vi "Controle_Manip_Main_GUI_Backup2.vi"() -> ()   [LabVIEW 2019] (continued)
          w103 = ""
          # "reset log file and \ncomment to empty"
          # "Build references arrays for real-time update of experiments' indicators"
          n40 = control-ref of="MasterPause"() -> (w60:refnum<vi>)
          n41 = control-ref of="MasterStop"() -> (w57:refnum<vi>)
          n42 = control-ref of="MasterPause"() -> (w58:refnum<vi>)
          n43 = control-ref of="MasterStop"() -> (w59:refnum<vi>)
          n44 = control-ref of="PausePolar"() -> ()  [unwired: 1 out]
          n45 = control-ref of="StopPolar"() -> ()  [unwired: 1 out]
          n46 = control-ref of="XY Intensity Map"() -> (w78:refnum<vi>)
          n47 = control-ref of="CCD 2D Image XY Map"() -> (w79:refnum<vi>)
          n48 = control-ref of="Expected (s)"() -> (w80:refnum<vi>)
          n49 = control-ref of="Elapsed (s)"() -> (w81:refnum<vi>)
          n50 = control-ref of="Scan X Readout (V)"() -> (w75:refnum<vi>)
          n51 = control-ref of="CCD 1D Spectrum XY Map"() -> (w77:refnum<vi>)
          n52 = control-ref of="Stop XY Map"() -> ()  [unwired: 1 out]
          n53 = control-ref of="Scan Y Readout (V)"() -> (w76:refnum<vi>)
          n54 = control-ref of="Scan Main Progess Bar"() -> (w72:refnum<vi>)
          n55 = control-ref of="Save XY Map"() -> (w74:refnum<vi>)
          n56 = control-ref of="Acquire XY Map"() -> (w73:refnum<vi>)
          n57 = control-ref of="KCube Shutter Device Reference"() -> (w90:refnum<vi>)
          n58 = control-ref of="RotStage Exc Angle Readout (°)"() -> (w85:refnum<vi>)
          n59 = control-ref of="RotStage Det Angle Readout (°)"() -> (w86:refnum<vi>)
          n60 = control-ref of="Polarisation 2D Image"() -> (w88:refnum<vi>)
          n61 = control-ref of="Pause XY Map"() -> ()  [unwired: 1 out]
          n62 = control-ref of="Polarisation 1D Spectrum"() -> (w87:refnum<vi>)
          n63 = control-ref of="Acquire Polarisation"() -> (w82:refnum<vi>)
          n64 = control-ref of="Scan Main Progess Bar"() -> (w84:refnum<vi>)
          n65 = control-ref of="Cnts"() -> (w70:refnum<vi>)
          n66 = control-ref of="Shutter Ctrls"() -> (w89:refnum<vi>)
          n67 = control-ref of="Save Polarisation"() -> (w83:refnum<vi>)
          n68 = Bundle("Scan Main Progess Bar"=w72, "Acquire XY Map"=w73, "MasterPause"=w58, "MasterStop"=w57, "Save XY Map"=w74, "Scan X Readout (V)"=w75, "Scan Y Readout (V)"=w76, "CCD 1D Spectrum XY Map"=w77, "XY Intensity Map"=w78, "CCD 2D Image XY Map"=w79, "Expected (s)"=w80, "Elapsed (s)"=w81, "Cnts"=w70) -> (→"Scan XY Map References":T31)  [unwired: 1 in]
          n69 = Bundle("Acquire Polarisation"=w82, "Save Polarisation"=w83, "MasterPause"=w60, "MasterStop"=w59, "Scan Main Progess Bar"=w84, "RotStage Exc Angle Readout (°)"=w85, "RotStage Det Angle Readout (°)"=w86, "Polarisation 1D Spectrum"=w87, "Polarisation 2D Image"=w88, "Shutter Ctrls"=w89, "KCube Shutter Device Reference"=w90) -> (→"Scan Polarisation References":T32)  [unwired: 1 in]
          n70 = control-ref of="Contrast Oscillations"() -> (w97:refnum<vi>)
          n71 = control-ref of="Acquire Contrast"() -> (w96:refnum<vi>)
          n72 = control-ref of="Contrast 1D Spectrum"() -> (w98:refnum<vi>)
          n73 = control-ref of="Save Contrast"() -> (w95:refnum<vi>)
          n74 = control-ref of="Att Pos X"() -> (w63:refnum<vi>)
          n75 = control-ref of="Att Pos Y"() -> (w62:refnum<vi>)
          n76 = control-ref of="Att Pos Z"() -> (w64:refnum<vi>)
          n77 = control-ref of="KCube Shutter Device Reference"() -> (w102:refnum<vi>)
          n78 = control-ref of="PZC Position Readout (usteps)"() -> (w101:refnum<vi>)
          n79 = control-ref of="Stop Contrast"() -> (w99:refnum<vi>)
          n80 = control-ref of="Scan Main Progess Bar"() -> (w94:refnum<vi>)
          n81 = control-ref of="Scan Y Readout (V)"() -> (w68:refnum<vi>)
          n82 = control-ref of="Scan X Readout (V)"() -> (w67:refnum<vi>)
          n83 = local write "NewVal"(FALSE ("NewVal")) -> ()
          n84 = control-ref of="Map Marker X Pos"() -> (w66:refnum<vi>)
          n85 = control-ref of="Map Marker Y Pos"() -> (w65:refnum<vi>)
          n86 = control-ref of="Pause Contrast"() -> (w100:refnum<vi>)
          n87 = control-ref of="Shutter Ctrls"() -> (w92:refnum<vi>)
          n88 = Bundle("Shutter Ctrls"=w92, "KCube Shutter Device Reference"=w102, "Scan Main Progess Bar"=w94, "PZC Position Readout (usteps)"=w101, "Pause Contrast"=w100, "Stop Contrast"=w99, "Contrast 1D Spectrum"=w98, "Contrast Oscillations"=w97, "Acquire Contrast"=w96, "Save Contrast"=w95) -> (→"Contrast References":T14)  [unwired: 1 in]
          n89 = Bundle("Scan Y Readout (V)"=w68, "Scan X Readout (V)"=w67, "Map Marker X Pos"=w66, "Map Marker Y Pos"=w65, "Att Pos Z"=w64, "Att Pos X"=w63, "Att Pos Y"=w62) -> (→"Location Parameters":T6)  [unwired: 1 in]
          n90 = local write "Log file"(w103) -> ()
          n91 = local write "Comment"(w103) -> ()
        }
        frame #3 {
          # "Get Experiment Graph Control numbers"
          n92 = control-ref of="Experiment Graph Controls"() -> (w107:refnum<vi>)
          n93 = property class="TabCtl (strict)"(reference=w107) -> ("Pages"=w105:refnum<vi>[])  [unwired: 1 in, 2 out]
          n94 = call "TabVisibility.vi"("Page Visible"=TRUE, "array"=w105, "MyfinalExpGraphCont"=T29."Absorption" ("Experiment Graph Controls")) -> ()  [unwired: 1 in]
        }
      }
    }
    frame #1 {
      # "Initialisation of all the devices?"
      # "Initialisation of devices connections"
      n95 = call "Initialisation prompt"() -> ("Yes please!"=w108:bool)  [unwired: 18 in, 1 out]
      "Initialise all devices?" <- w108
      n96 = case shown="True" w108 {
        frame False {
          # "Do not activate devices"
          n97 = control-ref of="Tab Objective Sample"() -> (w115:refnum<vi>)
          n98 = property on="Experimental parameters tab" class="TabCtl (strict)" props=["Pages", "Value"]() -> ("Pages"=w117:refnum<vi>[])  [unwired: 2 in, 3 out]
          n99 = property class="TabCtl (strict)"(reference=w115) -> ("Pages"=w113:refnum<vi>[])  [unwired: 1 in, 2 out]
          n100 = property on="Experiment Graph Controls" class="TabCtl (strict)" props=["Value", "Pages"]() -> ("Pages"=w119:refnum<vi>[])  [unwired: 2 in, 3 out]
          n101 = Array Size(array=w113) -> (size(s)=w114:i32)
          n102 = Array Size(array=w117) -> (size(s)=w116:i32)
          n103 = for {
            N: w116 -> [_]
            tunnel: w117 -> [w126]
            i -> [w124]
            n104 = Index Array(array=w126, index=w124) -> (element=w127:refnum<vi>)
            n105 = property class="Page"(reference=w127, "PageVis"=TRUE ("Page Visible")) -> ()  [unwired: 1 in, 2 out]
          }
          n106 = for {
            N: w114 -> [_]
            tunnel: w113 -> [w123]
            i -> [w122]
            n107 = Index Array(array=w123, index=w122) -> (element=w121:refnum<vi>)
            n108 = property class="Page"(reference=w121, "PageVis"=TRUE ("Page Visible")) -> ()  [unwired: 1 in, 2 out]
          }
          n109 = Array Size(array=w119) -> (size(s)=w118:i32)
          n110 = for {
            N: w118 -> [_]
            tunnel: w119 -> [w130]
            i -> [w128]
            n111 = Index Array(array=w130, index=w128) -> (element=w131:refnum<vi>)
            n112 = property class="Page"(reference=w131, "PageVis"=TRUE ("Page Visible")) -> ()  [unwired: 1 in, 2 out]
          }
          n113 = local read "Log file"() -> (w111:string)
          n114 = call "Write2LogFile.vi"("Add to log file"="Initialisation ...\nNo instruments activated.", "Log file before"=w111, "Checkbox"=FALSE) -> ("Log file after"=w112:string)
          n115 = local write "Log file"(w112) -> ()
        }
        frame True {
          # "Activate all the devices selected in the Settings tab"
          n116 = stacked-sequence {
            frame #0 {
              n117 = local read "ESP 301 On?"() -> (w140:bool)
              n118 = local read "ESP 300 On?"() -> (w141:bool)
              n119 = local read "PZC200 On?"() -> (w134:bool)
              n120 = local write "Scan Main Progess Bar"(u8 0 ("Scan Main Progess Bar")) -> ()
              n121 = local read "KCube Shutter On?"() -> (w138:bool)
              n122 = local read "KCubes Piezo On?"() -> (w137:bool)
              n123 = local read "Laser Comm On?"() -> (w132:bool)
              n124 = local read "Cryostation On?"() -> (w142:bool)
              n125 = local read "Attocubes On?"() -> (w143:bool)
              n126 = local read "PM16-120 On?"() -> (w135:bool)
              n127 = local read "LightField On?"() -> (w136:bool)
              n128 = local read "PicoHarp On?"() -> (w133:bool)
              n129 = local read "FSM 300 On?"() -> (w139:bool)
              n130 = global write "InstrumentsOn.vi" "ESP 301 On?"(w140) -> ()
              n131 = global write "InstrumentsOn.vi" "ESP 300 On?"(w141) -> ()
              n132 = global write "InstrumentsOn.vi" "PZC200 On?"(w134) -> ()
              n133 = global write "InstrumentsOn.vi" "Attocubes On?"(w143) -> ()
              n134 = global write "InstrumentsOn.vi" "Cryostation On?"(w142) -> ()
              n135 = global write "InstrumentsOn.vi" "PM16-120 On?"(w135) -> ()
              n136 = global write "InstrumentsOn.vi" "LightField On?"(w136) -> ()
              n137 = global write "InstrumentsOn.vi" "Laser Comm On?"(w132) -> ()
              n138 = global write "InstrumentsOn.vi" "KCubes Piezo On?"(w137) -> ()
              n139 = global write "InstrumentsOn.vi" "KCube Shutter On?"(w138) -> ()
              n140 = global write "InstrumentsOn.vi" "FSM 300 On?"(w139) -> ()
              n141 = global write "InstrumentsOn.vi" "PicoHarp On?"(w133) -> ()
            }
            frame #1 {
              # "LLTF"
              n142 = case shown="True" "LLTF On?" {
                frame False {
                }
                frame True {
                  n143 = Automation Open(Automation Refnum="xphyspecLib.IXPhySpec") -> (Automation Refnum=w163:refnum<k7>, error out=w162:errorcluster)  [unwired: 3 in]
                  n144 = local read "Excitation Wavelength (nm)"() -> (w153:dbl)
                  n145 = call "newinit.vi"("error in"=w162, "Automation Refnum"=w163) -> ("error out"=w159:errorcluster, "Detected?"=→"LLTF Detected?":bool, "xphyspecLib.IXPhySpec out"=w160:refnum<k7>)  [unwired: 7 in]
                  n146 = call "listandgetdeviceinterface.vi"("error in (no error)"=w159, "reference"=w160) -> ("LLTF error out"=→"LLTFDevice error out":errorcluster, "LLTFDevice Interface"=w155:refnum<k7>, "error out to close"=→"LLTF Error":errorcluster, "reference out to lose"=→"LLTF Reference":refnum<k7>)  [unwired: 6 in]
                  n147 = call "testmove.vi"("p_TargetWavelength"=w153, "reference"=w155) -> ("CurrentWavelength"=→"CurrentWL":dbl, "CurrentAngle"=→"CurrentAngle":dbl, "Device reference out"=→"LLTFDevice Interface":refnum<k7>, "Device moved"=→"Device moved":bool)  [unwired: 4 in, 2 out]
                  n148 = local read "Log file"() -> (w149:string)
                  n149 = call "Write2LogFile.vi"("Add to log file"="Initialise communication with PhotonEtc LLTF", "Log file before"=w149, "Checkbox"=FALSE) -> ("Log file after"=w148:string)
                  n150 = local write "Log file"(w148) -> ()
                }
              }
            }
            frame #2 {
              # "ESP 300: 1 Jobin Yvon 320 Monochromator"
              n151 = control-ref of="CCD 1D Spectrum Main  Cursor2WL 1 Mono 2"() -> (w167:refnum<vi>)
              n152 = control-ref of="CCD 1D Spectrum Main  Cursor2WL 2 Mono 2"() -> (w166:refnum<vi>)
              n153 = local read "ESP300 COM Port"() -> (w165:refnum<visa-resource-name>)
              n154 = case shown="True" "ESP 300 On?" {
                tunnel: [enum16{"Enabled", "Disabled", "Disabled&Grayed"}."Disabled&Grayed" ("Enum") enum16{"Enabled", "Disabled", "Disabled&Grayed"}."Enabled" ("Enum")] -> w169
                tunnel: w165 -> [w174 w177]
                frame False {
                  n155 = global write "InstrumentReferences.vi" "ESP300 COM Port"(w174) -> ()
                }
                frame True {
                  n156 = global write "InstrumentReferences.vi" "ESP300 COM Port"(w177) -> ()
                  n157 = control-ref of="Mono2 Velocity"() -> (w181:refnum<vi>)
                  n158 = control-ref of="Mono2 Motor Pos"() -> (w180:refnum<vi>)
                  n159 = call "subVI_Init&GetParams.vi"("Mono2 Pos"=w180, "Mono2 Velocity"=w181) -> ("Mono2 On"=w182:bool)  [unwired: 1 in]
                  n160 = local read "Log file"() -> (w186:string)
                  n161 = local write "Mono2 On"(w182) -> ()
                  n162 = call "Write2LogFile.vi"("Add to log file"="Initialise communication with ESP 300", "Log file before"=w186, "Checkbox"=FALSE) -> ("Log file after"=w185:string)
                  n163 = local write "Log file"(w185) -> ()
                  n164 = control-ref of="Mono2 Wavelength (nm)"() -> (w179:refnum<vi>)
                  n165 = property class="DigNum (strict)"(reference=w179, "DisabledEnum"=T28."Disabled and Grayed Out" ("Disabled")) -> ()  [unwired: 1 in, 2 out]
                }
              }
              n166 = control-ref of="Mono2 On"() -> (w170:refnum<vi>)
              n167 = control-ref of="Mono2 Wavelength (nm)"() -> (w171:refnum<vi>)
              n168 = control-ref of="Mono2 Motor Pos"() -> (w168:refnum<vi>)
              n169 = Build Array(w170, w171, w168, w167, w166) -> (w172:refnum<vi>[])
              n170 = call "Enable&Disable_Controls.vi"("Enum"=w169, "References"=w172) -> ()  [unwired: 1 in]
            }
            frame #3 {
              # "ESP 301: 2 rotation stages + 1 linear translation stage"
              n171 = case shown="True" "ESP 301 On?" {
                frame False {
                  n172 = control-ref of="Experiment Graph Controls"() -> (w190:refnum<vi>)
                  n173 = local read "Scan Polar AllParams"() -> (w202:refnum<vi>[])
                  n174 = property class="TabCtl (strict)"(reference=w190) -> ("Pages"=w194:refnum<vi>[])  [unwired: 1 in, 2 out]
                  n175 = property class="TabCtl (strict)"(reference=w190) -> ("Pages"=w191:refnum<vi>[])  [unwired: 1 in, 2 out]
                  n176 = call "Enable&Disable_Controls.vi"("Enum"=enum16{"Enabled", "Disabled", "Disabled&Grayed"}."Disabled&Grayed", "References"=w202) -> ()  [unwired: 1 in]
                  n177 = property on="Experimental parameters tab" class="TabCtl (strict)"() -> ("Pages"=w197:refnum<vi>[])  [unwired: 2 in, 2 out]
                  n178 = call "TabVisibility.vi"("Page Visible"=FALSE, "array"=w194, "MyfinalExpGraphCont"=T29."Polarisation Acquisition") -> ()  [unwired: 1 in]
                  n179 = call "TabVisibility.vi"("Page Visible"=FALSE, "array"=w191, "MyfinalExpGraphCont"=T29."Contrast Acquisition") -> ()  [unwired: 1 in]
                  n180 = local read "Scan Translation Coarse Ctrls"() -> (w196:refnum<vi>[])
                  n181 = Index Array(array=w197, index=2) -> (element=w204:refnum<vi>)
                  n182 = Index Array(array=w197, index=3) -> (element=w198:refnum<vi>)
                  n183 = property class="Page"(reference=w198, "PageVis"=FALSE ("Page Visible")) -> ()  [unwired: 1 in, 2 out]
                  n184 = property class="Page"(reference=w204, "PageVis"=FALSE ("Page Visible")) -> ()  [unwired: 1 in, 2 out]
                  n185 = call "Enable&Disable_Controls.vi"("Enum"=enum16{"Enabled", "Disabled", "Disabled&Grayed"}."Disabled&Grayed", "References"=w196) -> ()  [unwired: 1 in]
                }
                frame True {
                  n186 = stacked-sequence {
                    frame #0 {
                      n187 = local read "Log file"() -> (w209:string)
                      n188 = call "Write2LogFile.vi"("Add to log file"="Initialise communication with ESP 301", "Log file before"=w209, "Checkbox"=FALSE) -> ("Log file after"=w207:string)
                      n189 = local write "Log file"(w207) -> ()
                    }
                    frame #1 {
                      n190 = control-ref of="Experiment Graph Controls"() -> (w216:refnum<vi>)
                      n191 = property class="TabCtl (strict)"(reference=w216) -> ("Pages"=w217:refnum<vi>[])  [unwired: 1 in, 2 out]
                      n192 = property on="Experimental parameters tab" class="TabCtl (strict)"("Value"=T19."Polarisation" ("Experimental parameters tab")) -> ("Pages"=w222:refnum<vi>[])  [unwired: 2 in, 2 out]
                      n193 = property on="Experimental parameters tab" class="TabCtl (strict)"() -> ("Pages"=w229:refnum<vi>[])  [unwired: 2 in, 2 out]
                      n194 = property class="TabCtl (strict)"(reference=w216) -> ("Pages"=w220:refnum<vi>[])  [unwired: 1 in, 2 out]
                      n195 = call "TabVisibility.vi"("Page Visible"=TRUE, "array"=w217, "MyfinalExpGraphCont"=T29."Contrast Acquisition") -> ()  [unwired: 1 in]
                      n196 = Index Array(array=w222, index=3) -> (element=w225:refnum<vi>)
                      n197 = Index Array(array=w229, index=2) -> (element=w226:refnum<vi>)
                      n198 = call "TabVisibility.vi"("Page Visible"=TRUE, "array"=w220, "MyfinalExpGraphCont"=T29."Polarisation Acquisition") -> ()  [unwired: 1 in]
                      n199 = property class="Page"(reference=w226, "PageVis"=TRUE ("Page Visible")) -> ()  [unwired: 1 in, 2 out]
                      n200 = property class="Page"(reference=w225, "PageVis"=TRUE ("Page Visible")) -> ()  [unwired: 1 in, 2 out]
                      n201 = local read "Scan Translation Coarse Ctrls"() -> (w215:refnum<vi>[])
                      n202 = local read "Scan Polar AllParams"() -> (w213:refnum<vi>[])
                      n203 = call "Enable&Disable_Controls.vi"("Enum"=enum16{"Enabled", "Disabled", "Disabled&Grayed"}."Enabled", "References"=w215) -> ()  [unwired: 1 in]
                      n204 = call "Enable&Disable_Controls.vi"("Enum"=enum16{"Enabled", "Disabled", "Disabled&Grayed"}."Enabled", "References"=w213) -> ()  [unwired: 1 in]
                    }
                    frame #2 {
                      n205 = flat-sequence {
                        tunnel: [w236] -> w230
                        frame #0 {
                          w236 = refnum<visa-resource-name> "COM8" ("ESP 301 COM Port")
                          n206 = call "Close.vi"("VISA resource name"=w236) -> ()  [unwired: 10 in, 1 out]
                        }
                        frame #1 {
                          n207 = call "_Create Instrument Channel_libESP301.vi"("COM Port (1)"=u16 8) -> ()  [unwired: 8 in, 3 out]
                        }
                      }
                      n208 = call "Initialize.vi"("VISA resource name"=w230, "ID Query (True)"=TRUE, "Reset (False)"=FALSE ("ID Query (True)"), "Serial Link (RS232)"=enum16{"RS232", "USB"}."USB") -> ("VISA resource name out"=w231:refnum<visa-resource-name>, "error out"=w235:errorcluster)  [unwired: 5 in]
                      n209 = case shown="Default" w235 {
                        tunnel: w231 -> [_ _]
                        frame No Error {
                        }
                        frame Default {
                          w243 = FALSE ("ID Query (True)")
                          n210 = call "Connect Newport Instruments_libESP301.vi"() -> ("error (duplicate)"=w241:errorcluster, "VISA resource name (duplicate)"=w238:refnum<visa-resource-name>)  [unwired: 7 in, 3 out]
                          n211 = call "_Close Communications_libESP301.vi"("Instrument Channel"=w238, "error in (no error)"=w241) -> ("error out"=w240:errorcluster)  [unwired: 13 in]
                          n212 = call "Initialize.vi"("VISA resource name"=w238, "ID Query (True)"=w243, "Reset (False)"=w243, "error in (no error)"=w240, "Serial Link (RS232)"=enum16{"RS232", "USB"}."USB") -> ("VISA resource name out"=w239:refnum<visa-resource-name>)  [unwired: 4 in, 1 out]
                          n213 = local write "ESP 301 COM Port"(w239) -> ()
                        }
                      }
                      n214 = local write "ESP 301 COM Port"(w231) -> ()
                    }
                    frame #3 {
                      # "Initialise ESP301 communication\nand motor parameters & limits"
                      n215 = local read "ESP 301 COM Port"() -> (w244:refnum<visa-resource-name>)
                      n216 = for {
                        N: 3 -> [_]
                        tunnel: w244 -> [w257]
                        tunnel: [w256] -> _
                        i -> [w247]
                        n217 = Increment(x=w247) -> (x+1=w246:i32)
                        n218 = call "Get Left Travel Limit.vi"("Axis (1)"=w246, "VISA resource name"=w257) -> ("Left Travel Limit (units)"=w253:dbl, "VISA resource name out"=w260:refnum<visa-resource-name>)  [unwired: 3 in, 1 out]
                        n219 = call "Get Right Travel Limit.vi"("Axis (1)"=w246, "VISA resource name"=w260) -> ("Right Travel Limit (units)"=w252:dbl, "VISA resource name out"=w259:refnum<visa-resource-name>)  [unwired: 3 in, 1 out]
                        n220 = call "Get Velocity.vi"("Axis (1)"=w246, "VISA resource name"=w259) -> ("Velocity (units/s)"=w251:dbl, "VISA resource name out"=w258:refnum<visa-resource-name>)  [unwired: 3 in, 1 out]
                        n221 = call "Read Actual Position.vi"("Axis (1)"=w246, "VISA resource name"=w258) -> ("Position (units)"=w248:dbl, "VISA resource name out"=w255:refnum<visa-resource-name>)  [unwired: 3 in, 1 out]
                        n222 = call "Get Maximum Velocity.vi"("Axis (1)"=w246, "VISA resource name"=w255) -> ("Maximum Velocity (units/s)"=w250:dbl, "VISA resource name out"=w254:refnum<visa-resource-name>)  [unwired: 3 in, 1 out]
                        n223 = call "Get Motor Power Status.vi"("Axis (1)"=w246, "VISA resource name"=w254) -> ("Power Status"=w249:bool, "VISA resource name out"=w256:refnum<visa-resource-name>)  [unwired: 3 in, 1 out]
                        n224 = case shown="1" w246 {
                          tunnel: w253 -> [_ w266 w272 w278]
                          tunnel: w252 -> [_ w265 w271 w277]
                          tunnel: w251 -> [_ w264 w270 w275]
                          tunnel: w250 -> [_ w263 w268 w276]
                          tunnel: w249 -> [_ w262 w267 w273]
                          tunnel: w248 -> [_ w261 w269 w274]
                          frame 0, Default {
                          }
                          frame 1 {
                            # "Translation stage"
                            n225 = property on="Newport Linear Translation Stage Position (mm)" class="DigNum (strict)"("Minimum"=w266, "Maximum"=w265) -> ()  [unwired: 2 in, 2 out]
                            n226 = local write "Newport Linear Translation Stage Velocity (mm/s)"(w264) -> ()
                            n227 = local write "Newport Linear Translation Stage Position Readout (mm)"(w261) -> ()
                            n228 = property on="Newport Linear Translation Stage Velocity (mm/s)" class="DigNum (strict)"("Maximum"=w263) -> ()  [unwired: 2 in, 2 out]
                            n229 = local write "Motor LinT On?"(w262) -> ()
                          }
                          frame 2 {
                            # "RotStage Det"
                            n230 = property on="RotStage Det Angle (°)" class="DigNum (strict)"("Maximum"=w272, "Minimum"=w271) -> ()  [unwired: 2 in, 2 out]
                            n231 = local write "RotStage Det Velocity (°/s)"(w270) -> ()
                            n232 = property on="RotStage Det Velocity (°/s)" class="DigNum (strict)"("Maximum"=w268) -> ()  [unwired: 2 in, 2 out]
                            n233 = local write "RotStage Det Angle Readout (°)"(w269) -> ()
                            n234 = local write "Motor RotStage Det On?"(w267) -> ()
                          }
                          frame 3 {
                            # "RotStage Exc"
                            n235 = property on="RotStage Exc Angle (°)" class="DigNum (strict)"("Maximum"=w278, "Minimum"=w277) -> ()  [unwired: 2 in, 2 out]
                            n236 = local write "RotStage Exc Velocity (°/s)"(w275) -> ()
                            n237 = property on="RotStage Exc Velocity (°/s)" class="DigNum (strict)"("Maximum"=w276) -> ()  [unwired: 2 in, 2 out]
                            n238 = local write "RotStage Exc Angle Readout (°)"(w274) -> ()
                            n239 = local write "Motor RotStage Exc On?"(w273) -> ()
                          }
                        }
                      }
                    }
                    frame #4 {
                      n240 = local read "ESP 301 COM Port"() -> (w279:refnum<visa-resource-name>)
                      n241 = call "Get Motor Power Status.vi"("Axis (1)"=1, "VISA resource name"=w279) -> ("error out"=w286:errorcluster, "Power Status"=w282:bool, "VISA resource name out"=w287:refnum<visa-resource-name>)  [unwired: 3 in]
                      n242 = local write "Motor LinT On?"(w282) -> ()
                      n243 = call "Get Motor Power Status.vi"("error in (no error)"=w286, "Axis (1)"=2, "VISA resource name"=w287) -> ("error out"=w289:errorcluster, "Power Status"=w280:bool, "VISA resource name out"=w288:refnum<visa-resource-name>)  [unwired: 2 in]
                      n244 = local write "Motor RotStage Exc On?"(w280) -> ()
                      n245 = call "Get Motor Power Status.vi"("error in (no error)"=w289, "Axis (1)"=3, "VISA resource name"=w288) -> ("error out"=w290:errorcluster, "Power Status"=w281:bool)  [unwired: 2 in, 1 out]
                      n246 = local write "Motor RotStage Det On?"(w281) -> ()
                      n247 = local write "ESP 301 Error"(w290) -> ()
                    }
                  }
                }
              }
            }
            frame #4 {
              # "Advance progress bar"
              n248 = local write "Scan Main Progess Bar"(u8 5 ("Scan Main Progess Bar")) -> ()
            }
            frame #5 {
              # "LightField: Monochromator SpectraPro HRS-500 + CCD Pixis"
              n249 = case shown="True" "LightField On?" {
                frame False {
                  n250 = control-ref of="Grating"() -> (w306:refnum<vi>)
                  n251 = control-ref of="Center Wavelength (nm)"() -> (w308:refnum<vi>)
                  n252 = local read "PicoHarp On?"() -> (w314:bool)
                  n253 = local read "ESP 300 On?"() -> (w315:bool)
                  n254 = control-ref of="Accumulations"() -> (w311:refnum<vi>)
                  n255 = control-ref of="CCD ROI"() -> (w310:refnum<vi>)
                  n256 = control-ref of="Exposure Time (ms)"() -> (w309:refnum<vi>)
                  n257 = control-ref of="Exit mirror"() -> (w307:refnum<vi>)
                  n258 = And(x=w315, y=w314) -> (x .and. y?=w313:bool)
                  n259 = case shown="False" w313 {
                    frame False {
                      n260 = control-ref of="Experiment Graph Controls"() -> (w317:refnum<vi>)
                      n261 = property class="TabCtl (strict)"(reference=w317) -> ("Pages"=w319:refnum<vi>[])  [unwired: 1 in, 2 out]
                      n262 = call "TabVisibility.vi"("Page Visible"=FALSE, "array"=w319, "MyfinalExpGraphCont"=T29."Spectrum Acquisition") -> ()  [unwired: 1 in]
                    }
                    frame True {
                      n263 = control-ref of="Experiment Graph Controls"() -> (w321:refnum<vi>)
                      n264 = property class="TabCtl (strict)"(reference=w321) -> ("Pages"=w323:refnum<vi>[])  [unwired: 1 in, 2 out]
                      n265 = call "TabVisibility.vi"("Page Visible"=TRUE, "array"=w323, "MyfinalExpGraphCont"=T29."Spectrum Acquisition") -> ()  [unwired: 1 in]
                    }
                  }
                  n266 = Build Array(w308, w307, w306, w311, w310, w309) -> (w312:refnum<vi>[])
                  n267 = call "Enable&Disable_Controls.vi"("Enum"=enum16{"Enabled", "Disabled", "Disabled&Grayed"}."Disabled&Grayed", "References"=w312) -> ()  [unwired: 1 in]
                  n268 = control-ref of="Experiment Graph Controls"() -> (w304:refnum<vi>)
                  n269 = control-ref of="Experiment Graph Controls"() -> (w299:refnum<vi>)
                  n270 = control-ref of="Experiment Graph Controls"() -> (w298:refnum<vi>)
                  n271 = property class="TabCtl (strict)"(reference=w304) -> ("Pages"=w302:refnum<vi>[])  [unwired: 1 in, 2 out]
                  n272 = property class="TabCtl (strict)"(reference=w299) -> ("Pages"=w301:refnum<vi>[])  [unwired: 1 in, 2 out]
                  n273 = property class="TabCtl (strict)"(reference=w298) -> ("Pages"=w296:refnum<vi>[])  [unwired: 1 in, 2 out]
                  n274 = call "TabVisibility.vi"("Page Visible"=FALSE, "array"=w302, "MyfinalExpGraphCont"=T29."Intensity Map Acquisition") -> ()  [unwired: 1 in]
                  n275 = call "TabVisibility.vi"("Page Visible"=FALSE, "array"=w301, "MyfinalExpGraphCont"=T29."Polarisation Acquisition") -> ()  [unwired: 1 in]
                  n276 = call "TabVisibility.vi"("Page Visible"=FALSE, "array"=w296, "MyfinalExpGraphCont"=T29."Contrast Acquisition") -> ()  [unwired: 1 in]
                }
                frame True {
                  n277 = stacked-sequence {
                    seq-local: [_ _ "uPL" ("ExperimentName") _ _ _ _] -> [_ _ _ w354 _ _ _]
                    seq-local: [_ _ w348 _ _ _ _] -> [_ _ _ w355 _ _ _]
                    seq-local: [_ _ w347 _ _ _ _] -> [_ _ _ w353 _ _ _]
                    seq-local: [_ _ _ w352 _ _ _] -> [_ _ _ _ w364 _ _]
                    seq-local: [_ _ _ w351 _ _ _] -> [_ _ _ _ w363 _ _]
                    seq-local: [_ _ _ _ w358 _ _] -> [_ _ _ _ _ w371 _]
                    seq-local: [_ _ _ _ w359 _ _] -> [_ _ _ _ _ w372 _]
                    seq-local: [_ _ _ _ w357 _ _] -> [_ _ _ _ _ w370 _]
                    frame #0 {
                      n278 = control-ref of="Grating"() -> (w326:refnum<vi>)
                      n279 = control-ref of="Center Wavelength (nm)"() -> (w328:refnum<vi>)
                      n280 = control-ref of="Accumulations"() -> (w331:refnum<vi>)
                      n281 = control-ref of="CCD ROI"() -> (w330:refnum<vi>)
                      n282 = control-ref of="Exposure Time (ms)"() -> (w329:refnum<vi>)
                      n283 = control-ref of="Exit mirror"() -> (w327:refnum<vi>)
                      n284 = local read "Log file"() -> (w334:string)
                      n285 = Build Array(w328, w327, w326, w331, w330, w329) -> (w332:refnum<vi>[])
                      n286 = call "Write2LogFile.vi"("Add to log file"="Launching LightField (~ 20 s)", "Log file before"=w334, "Checkbox"=FALSE) -> ("Log file after"=w335:string)
                      n287 = call "Enable&Disable_Controls.vi"("Enum"=enum16{"Enabled", "Disabled", "Disabled&Grayed"}."Enabled", "References"=w332) -> ()  [unwired: 1 in]
                      n288 = local write "Log file"(w335) -> ()
                    }
                    frame #1 {
                      n289 = control-ref of="Experiment Graph Controls"() -> (w337:refnum<vi>)
                      n290 = control-ref of="Experimental parameters tab"() -> (w341:refnum<vi>)
                      n291 = property class="TabCtl (strict)"(reference=w337) -> ("Pages"=w339:refnum<vi>[])  [unwired: 1 in, 2 out]
                      n292 = property class="TabCtl (strict)"(reference=w341, "Value"=T19."Monochromators & CCD") -> ("Pages"=w344:refnum<vi>[])  [unwired: 1 in, 2 out]
                      n293 = call "TabVisibility.vi"("Page Visible"=TRUE, "array"=w339, "MyfinalExpGraphCont"=T29."Spectrum Acquisition") -> ()  [unwired: 1 in]
                      n294 = Index Array(array=w344, index=0) -> (element=w345:refnum<vi>)
                      n295 = property class="Page"(reference=w345, "PageVis"=TRUE ("Page Visible")) -> ()  [unwired: 1 in, 2 out]
                    }
                    frame #2 {
                      n296 = call "LFA_Initialize.vi"("Is Visible?"="LF Visible") -> ("error out"=w348:errorcluster, "LightField Automation out"=w347:refnum<class "LightField Automation.lvclass">)  [unwired: 9 in]
                    }
                    frame #3 {
                      n297 = local write "Scan Main Progess Bar"(u8 15 ("Scan Main Progess Bar")) -> ()
                      n298 = call "Exp_SetExperiment.vi"("error in (no error)"=w355, "ExperimentName"=w354, "LightField Automation in"=w353) -> ("error out"=w352:errorcluster, "LightField Automation out"=w351:refnum<class "LightField Automation.lvclass">)  [unwired: 7 in]
                    }
                    frame #4 {
                      n299 = local read "Log file"() -> (w362:string)
                      n300 = call "Write2LogFile.vi"("Add to log file"="Getting parameters", "Log file before"=w362, "Checkbox"=FALSE) -> ("Log file after"=w361:string)
                      n301 = local write "Log file"(w361) -> ()
                      n302 = call "Exp_CCD_GetExposureTime.vi"("error in (no error)"=w364, "LightField Automation in"=w363) -> ("error out"=w358:errorcluster, "Exposure Time (s)"=w357:dbl, "LightField Automation out"=w359:refnum<class "LightField Automation.lvclass">)  [unwired: 7 in]
                    }
                    frame #5 {
                      n303 = call "Exp_CCD_GetTemperature.vi"("error in (no error)"=w371, "LightField Automation in"=w372) -> ("error out"=w375:errorcluster, "Temperature (°C)"=→"CCD T° :":dbl, "LightField Automation out"=w374:refnum<class "LightField Automation.lvclass">)  [unwired: 7 in]
                      n304 = call "spec_GetGratings.vi"("error in (no error)"=w375, "LightField Automation in"=w374) -> ("error out"=w383:errorcluster, "Current Grating"=w377:string, "LightField Automation out"=w384:refnum<class "LightField Automation.lvclass">)  [unwired: 6 in, 1 out]
                      n305 = call "spec_GetCenterWavelength.vi"("error in (no error)"=w383, "LightField Automation in"=w384) -> ("error out"=w381:errorcluster, "Center Wavelength"=w378:dbl, "LightField Automation out"=w380:refnum<class "LightField Automation.lvclass">)  [unwired: 7 in]
                      n306 = local write "Grating"(w377) -> ()
                      n307 = call "spec_getCalibration.vi"("error in (no error)"=w381, "LightField Automation in"=w380) -> ("error out"=w368:errorcluster, "ColumnCalibration"=→"Wavelength calibration":dbl[], "LightField Automation out"=w369:refnum<class "LightField Automation.lvclass">)  [unwired: 7 in]
                      n308 = call "spec_GetOpticalExitPort.vi"("error in (no error)"=w368, "LightField Automation in"=w369) -> ("error out"=w367:errorcluster, "Exit Port Location"=w366:T33, "LightField Automation out"=w365:refnum<class "LightField Automation.lvclass">)  [unwired: 7 in]
                      n309 = local write "Center Wavelength (nm)"(w378) -> ()
                      n310 = global write "InstrumentReferences.vi" "LightField Automation out"(w365) -> ()
                      n311 = local write "LightField Automation out"(w365) -> ()
                      n312 = local write "LightField Automation error out"(w367) -> ()
                      n313 = local write "Exit mirror"(w366) -> ()
                      n314 = Multiply(x=w370, y=1000.0) -> (x*y=w379:dbl)
                      n315 = local write "Exposure Time (ms)"(w379) -> ()
                      n316 = local write "Acq Time (ms)"(w379) -> ()
                    }
                    frame #6 {
                      n317 = local write "Scan Main Progess Bar"(u8 35 ("Scan Main Progess Bar")) -> ()
                    }
                  }
                }
              }
            }
            frame #6 {
              # "Thorlabs USB photodiode"
              n318 = case shown="True" "PM16-120 On?" {
                frame False {
                  n319 = property on="Excitation Power (uW)" class="DigNum (strict)"("Label.BG Color"=u32 16711680 ("Label.Colors:BG Color")) -> ()  [unwired: 2 in, 2 out]
                }
                frame True {
                  w389 = refnum<visa-resource-name> "USB0::0x1313::0x807B::190927109::INSTR" ("instrument handle")
                  # "Initialise powermeter"
                  n320 = call <instrlib>:"TLPM Find Resources.vi"("instrument handle"=w389) -> ("error out"=w394:errorcluster, "Resource Count"=w396:u32)  [unwired: 8 in, 1 out]
                  n321 = property on="Excitation Power (uW)" class="DigNum (strict)"("Blinking"=FALSE) -> ()  [unwired: 2 in, 2 out]
                  n322 = Greater Or Equal?(x=w396, y=1) -> (x >= y?=w395:bool)
                  n323 = case shown="True" w395 {
                    tunnel: w394 -> [_ w409]
                    tunnel: w389 -> [w401 w402]
                    frame False {
                      w400 = FALSE ("ID Query (Do Query)")
                      n324 = call <instrlib>:"TLPM Initialize.vi"("Reset Device (Reset Device)"=w400, "ID Query (Do Query)"=w400, "resource name"=w401) -> ("error out"=w398:errorcluster, "instrument handle out"=w399:refnum<visa-resource-name>)  [unwired: 7 in]
                      n325 = local write "Photodiode handle out"(w399) -> ()
                      n326 = local write "Photodiode error out"(w398) -> ()
                    }
                    frame True {
                      w408 = FALSE ("Reset Device (Reset Device)")
                      # "Select first Device\n(Device Index 0)"
                      n327 = call <instrlib>:"TLPM Get Resource Name.vi"("error in (no error)"=w409, "Index (0)"=u32 0) -> ("error out"=w407:errorcluster)  [unwired: 7 in, 2 out]
                      n328 = local write "Photodiode Status"(TRUE) -> ()
                      n329 = call <instrlib>:"TLPM Initialize.vi"("error in (no error)"=w407, "Reset Device (Reset Device)"=w408, "ID Query (Do Query)"=w408, "resource name"=w402) -> ("error out"=w404:errorcluster, "instrument handle out"=w405:refnum<visa-resource-name>)  [unwired: 6 in]
                      n330 = local write "Photodiode handle out"(w405) -> ()
                      n331 = local write "Photodiode error out"(w404) -> ()
                    }
                  }
                  n332 = local read "Log file"() -> (w393:string)
                  n333 = call "Write2LogFile.vi"("Add to log file"="Initialise communication with Photodiode", "Log file before"=w393, "Checkbox"=FALSE) -> ("Log file after"=w392:string)
                  n334 = local write "Log file"(w392) -> ()
                }
              }
            }
            frame #7 {
              # "448.3nm Laser Diode + Temp Controller & Driver"
              n335 = case shown="True" "Laser Comm On?" {
                frame False {
                  w411 = FALSE ("Visible")
                  n336 = property on="TEC Output" class="Bool (strict)"("Visible"=w411) -> ()  [unwired: 2 in, 2 out]
                  n337 = property on="TEC Temperature" class="DigNum (strict)"("Visible"=w411) -> ()  [unwired: 2 in, 2 out]
                  n338 = property on="Laser Diode Current Set" class="Slide (strict)"("Visible"=w411) -> ()  [unwired: 2 in, 2 out]
                  n339 = property on="Laser on? Control" class="Bool (strict)"("Visible"=w411) -> ()  [unwired: 2 in, 2 out]
                }
                frame True {
                  n340 = local read "Log file"() -> (w415:string)
                  n341 = call "Write2LogFile.vi"("Add to log file"="Initialise communication with Laser Driver", "Log file before"=w415, "Checkbox"=FALSE) -> ("Log file after"=w414:string)
                  n342 = local write "Log file"(w414) -> ()
                  n343 = call "LaserDiodeInit.vi"("resource name"=refnum<visa-resource-name> "USB0::0x1313::0x804F::M00549740::INSTR" ("Diode Driver COM")) -> ("Diode Driver Error"=w420:errorcluster, "Temperature"=w417:dbl, "TEC Output"=w419:bool, "resource out"=→"DDE":refnum<visa-resource-name>, "LD Output"=w418:bool, "Serial Number"=→"Serial Number":string)
                  n344 = local write "Laser on?"(w418) -> ()
                  n345 = local write "Laser on? Control"(w418) -> ()
                  n346 = local write "TEC Output"(w419) -> ()
                  n347 = local write "TEC Temperature"(w417) -> ()
                  n348 = local write "Diode Driver Error"(w420) -> ()
                  n349 = property on="Laser Diode Current Set" class="Slide (strict)"("Visible"=w419) -> ()  [unwired: 2 in, 2 out]
                  n350 = property on="Laser Safety" class="Ring (strict)"("Visible"=w419) -> ()  [unwired: 2 in, 2 out]
                  n351 = property on="Laser on? Control" class="Bool (strict)"("Visible"=w419) -> ()  [unwired: 2 in, 2 out]
                }
              }
            }
            frame #8 {
              # "Excitation wavelength"
              n352 = disable-structure shown="Enabled" {
                disable-tunnel: [w426 458.3] -> w425
                frame Disabled {
                  n353 = call "PromptUserWavelength_DefautValue.vi"() -> ("Wavelength"=w426:dbl)  [unwired: 17 in, 2 out]
                }
                frame Enabled {
                }
              }
              n354 = call "nm2WL.vi"("Wavelength (380 - 780)"=w425) -> ("Color"=w423:u32, "Out Of Range"=w424:bool)
              n355 = case shown="False" w424 {
                tunnel: w423 -> [w431 _]
                frame False {
                  # "set laser color"
                  n356 = Bundle("Color"=w431, "Color"=w431) -> (w430:cluster{"Color":u32, "Color":u32})  [unwired: 1 in]
                  n357 = Bundle(u32 16777216, u32 16777216) -> (w429:cluster{u32, u32})  [unwired: 1 in]
                  n358 = Build Array(w429, w430) -> (w428:cluster{"Color":u32, "Color":u32}[])
                  n359 = property on="Laser on?" class="Bool (strict)"("Colors [4]"=w428) -> ()  [unwired: 2 in, 2 out]
                }
                frame True {
                }
              }
              n360 = local write "Excitation Wavelength (nm)"(w425) -> ()
            }
            frame #9 {
              # "Advancec progress bar"
              n361 = local write "Scan Main Progess Bar"(u8 50 ("Scan Main Progess Bar")) -> ()
            }
            frame #10 {
              # "FSM"
              n362 = local read "FSM 300 On?"() -> (w435:bool)
              n363 = case shown="True" w435 {
                frame True {
                  n364 = stacked-sequence {
                    frame #0 {
                      n365 = local read "Log file"() -> (w439:string)
                      n366 = call "Write2LogFile.vi"("Add to log file"="Initialise communication with FSM", "Log file before"=w439, "Checkbox"=FALSE) -> ("Log file after"=w438:string)
                      n367 = local write "Log file"(w438) -> ()
                    }
                    frame #1 {
                      n368 = control-ref of="Experiment Graph Controls"() -> (w440:refnum<vi>)
                      n369 = property on="Experimental parameters tab" class="TabCtl (strict)"("Value"=T19."Steering mirror" ("Experimental parameters tab")) -> ("Pages"=w448:refnum<vi>[])  [unwired: 2 in, 2 out]
                      n370 = property class="TabCtl (strict)"(reference=w440) -> ("Pages"=w442:refnum<vi>[])  [unwired: 1 in, 2 out]
                      n371 = Index Array(array=w448, index=1) -> (element=w446:refnum<vi>)
                      n372 = property class="Page"(reference=w446, "PageVis"=TRUE ("Page Visible")) -> ()  [unwired: 1 in, 2 out]
                      n373 = call "TabVisibility.vi"("Page Visible"=TRUE, "array"=w442, "MyfinalExpGraphCont"=T29."Intensity Map Acquisition" ("Experiment Graph Controls")) -> ()  [unwired: 1 in]
                    }
                    frame #2 {
                      w453 = 10.0 ("maximum value")
                      w455 = 10.0 ("maximum value")
                      n374 = local read "FSM Y Axis"() -> (w451:tag)
                      n375 = local read "FSM X Axis"() -> (w454:tag)
                      n376 = Negate(x=w455) -> (-x=w456:dbl)
                      n377 = Negate(x=w453) -> (-x=w452:dbl)
                      n378 = call-poly <vilib>:"DAQmx Create Virtual Channel.vi"("maximum value"=w455, "minimum value"=w456, "physical channels"=w454) -> ("task out"=→"FSM X Task":refnum<k21>)  [unwired: 11 in, 1 out]
                      n379 = call-poly <vilib>:"DAQmx Create Virtual Channel.vi"("maximum value"=w453, "minimum value"=w452, "physical channels"=w451) -> ("task out"=→"FSM Y Task":refnum<k21>)  [unwired: 11 in, 1 out]
                    }
                  }
                }
                frame False {
                  n380 = control-ref of="Experiment Graph Controls"() -> (w458:refnum<vi>)
                  n381 = property on="Experimental parameters tab" class="TabCtl (strict)"() -> ("Pages"=w464:refnum<vi>[])  [unwired: 2 in, 2 out]
                  n382 = property class="TabCtl (strict)"(reference=w458) -> ("Pages"=w460:refnum<vi>[])  [unwired: 1 in, 2 out]
                  n383 = Index Array(array=w464, index=1) -> (element=w462:refnum<vi>)
                  n384 = call "TabVisibility.vi"("Page Visible"=FALSE, "array"=w460, "MyfinalExpGraphCont"=T29."Intensity Map Acquisition") -> ()  [unwired: 1 in]
                  n385 = property class="Page"(reference=w462, "PageVis"=FALSE ("Page Visible")) -> ()  [unwired: 1 in, 2 out]
                }
              }
            }
            frame #11 {
              # "Set all graph styles according to CCD Acq Mode: Spectrum or 2D Image"
              n386 = local read "Acq Mode"() -> (w465:T3)
              n387 = case shown="\"Image\"" w465 {
                frame "Image" {
                  w487 = TRUE
                  w486 = FALSE
                  n388 = property on="CCD 2D Image Main" class="IntGraph (strict)"("Visible"=w487) -> ()  [unwired: 2 in, 2 out]
                  n389 = property on="CCD 2D Image XY Map" class="IntGraph (strict)"("Visible"=w487) -> ()  [unwired: 2 in, 2 out]
                  n390 = property on="CCD 1D Spectrum XY Map" class="WFGraph (strict)"("Visible"=w486) -> ()  [unwired: 2 in, 2 out]
                  n391 = property on="CCD 1D Spectrum Main" class="XYGraph (strict)"("Visible"=w486) -> ()  [unwired: 2 in, 2 out]
                }
                frame "Spectrum" {
                  w488 = FALSE
                  w489 = TRUE
                  n392 = property on="CCD 2D Image Main" class="IntGraph (strict)"("Visible"=w488) -> ()  [unwired: 2 in, 2 out]
                  n393 = property on="CCD 2D Image XY Map" class="IntGraph (strict)"("Visible"=w488) -> ()  [unwired: 2 in, 2 out]
                  n394 = property on="CCD 1D Spectrum XY Map" class="WFGraph (strict)"("Visible"=w489) -> ()  [unwired: 2 in, 2 out]
                  n395 = property on="CCD 1D Spectrum Main" class="XYGraph (strict)"("Visible"=w489) -> ()  [unwired: 2 in, 2 out]
                }
                frame "APD 1" {
                  w490 = FALSE
                  w491 = TRUE
                  n396 = property on="CCD 2D Image Main" class="IntGraph (strict)"("Visible"=w490) -> ()  [unwired: 2 in, 2 out]
                  n397 = property on="CCD 2D Image XY Map" class="IntGraph (strict)"("Visible"=w490) -> ()  [unwired: 2 in, 2 out]
                  n398 = property on="CCD 1D Spectrum XY Map" class="WFGraph (strict)"("Visible"=w491) -> ()  [unwired: 2 in, 2 out]
                  n399 = property on="CCD 1D Spectrum Main" class="XYGraph (strict)"("Visible"=w491) -> ()  [unwired: 2 in, 2 out]
                }
                frame "APD 2" {
                  w492 = FALSE
                  w493 = TRUE
                  n400 = property on="CCD 2D Image Main" class="IntGraph (strict)"("Visible"=w492) -> ()  [unwired: 2 in, 2 out]
                  n401 = property on="CCD 2D Image XY Map" class="IntGraph (strict)"("Visible"=w492) -> ()  [unwired: 2 in, 2 out]
                  n402 = property on="CCD 1D Spectrum XY Map" class="WFGraph (strict)"("Visible"=w493) -> ()  [unwired: 2 in, 2 out]
                  n403 = property on="CCD 1D Spectrum Main" class="XYGraph (strict)"("Visible"=w493) -> ()  [unwired: 2 in, 2 out]
                }
                frame "APD 1+2" {
                  w494 = FALSE
                  w495 = TRUE
                  n404 = property on="CCD 2D Image Main" class="IntGraph (strict)"("Visible"=w494) -> ()  [unwired: 2 in, 2 out]
                  n405 = property on="CCD 2D Image XY Map" class="IntGraph (strict)"("Visible"=w494) -> ()  [unwired: 2 in, 2 out]
                  n406 = property on="CCD 1D Spectrum XY Map" class="WFGraph (strict)"("Visible"=w495) -> ()  [unwired: 2 in, 2 out]
                  n407 = property on="CCD 1D Spectrum Main" class="XYGraph (strict)"("Visible"=w495) -> ()  [unwired: 2 in, 2 out]
                }
              }
              n408 = case shown="\"Spectrum\", Default" w465 {
                frame "Image" {
                  n409 = control-ref of="Experiment Graph Controls"() -> (w468:refnum<vi>)
                  n410 = property class="TabCtl (strict)"(reference=w468) -> ("Pages"=w469:refnum<vi>[])  [unwired: 1 in, 2 out]
                  n411 = call "TabVisibility.vi"("Page Visible"=FALSE, "array"=w469, "MyfinalExpGraphCont"=T29."Spectrum Acquisition") -> ()  [unwired: 1 in]
                }
                frame "Spectrum", Default {
                  n412 = control-ref of="Experiment Graph Controls"() -> (w471:refnum<vi>)
                  n413 = property class="TabCtl (strict)"(reference=w471) -> ("Pages"=w473:refnum<vi>[])  [unwired: 1 in, 2 out]
                  n414 = call "TabVisibility.vi"("Page Visible"=FALSE, "array"=w473, "MyfinalExpGraphCont"=T29."APDs Acquisition") -> ()  [unwired: 1 in]
                }
                frame "APD 1" {
                  n415 = control-ref of="Experiment Graph Controls"() -> (w475:refnum<vi>)
                  n416 = property class="TabCtl (strict)"(reference=w475) -> ("Pages"=w477:refnum<vi>[])  [unwired: 1 in, 2 out]
                  n417 = call "TabVisibility.vi"("Page Visible"=TRUE, "array"=w477, "MyfinalExpGraphCont"=T29."APDs Acquisition") -> ()  [unwired: 1 in]
                }
                frame "APD 2" {
                  n418 = control-ref of="Experiment Graph Controls"() -> (w479:refnum<vi>)
                  n419 = property class="TabCtl (strict)"(reference=w479) -> ("Pages"=w481:refnum<vi>[])  [unwired: 1 in, 2 out]
                  n420 = call "TabVisibility.vi"("Page Visible"=TRUE, "array"=w481, "MyfinalExpGraphCont"=T29."APDs Acquisition") -> ()  [unwired: 1 in]
                }
                frame "APD 1+2" {
                  n421 = control-ref of="Experiment Graph Controls"() -> (w483:refnum<vi>)
                  n422 = property class="TabCtl (strict)"(reference=w483) -> ("Pages"=w485:refnum<vi>[])  [unwired: 1 in, 2 out]
                  n423 = call "TabVisibility.vi"("Page Visible"=TRUE, "array"=w485, "MyfinalExpGraphCont"=T29."APDs Acquisition") -> ()  [unwired: 1 in]
                }
              }
            }
            frame #12 {
              # "KCubes: 1 Shutter + 3 Piezos for XYZ microscope objective"
              n424 = stacked-sequence {
                frame #0 {
                  # "Shutter"
                  n425 = case shown="True" "KCube Shutter On?" {
                    frame False {
                      n426 = control-ref of="Experimental parameters tab"() -> (w501:refnum<vi>)
                      n427 = property class="TabCtl (strict)"(reference=w501) -> ("Pages"=w499:refnum<vi>[])  [unwired: 1 in, 2 out]
                      n428 = Index Array(array=w499, index=5) -> (element=w498:refnum<vi>)
                      n429 = property class="Page"(reference=w498, "PageVis"=FALSE ("Page Visible")) -> ()  [unwired: 1 in, 2 out]
                    }
                    frame True {
                      n430 = stacked-sequence {
                        frame #0 {
                          n431 = local read "Log file"() -> (w505:string)
                          n432 = call "Write2LogFile.vi"("Add to log file"="Initialise communication with Shutter", "Log file before"=w505, "Checkbox"=FALSE) -> ("Log file after"=w504:string)
                          n433 = local write "Log file"(w504) -> ()
                        }
                        frame #1 {
                          n434 = control-ref of="Experimental parameters tab"() -> (w511:refnum<vi>)
                          n435 = property class="TabCtl (strict)"(reference=w511, "Value"=T19."Shutter options") -> ("Pages"=w509:refnum<vi>[])  [unwired: 1 in, 2 out]
                          n436 = Index Array(array=w509, index=5) -> (element=w508:refnum<vi>)
                          n437 = property class="Page"(reference=w508, "PageVis"=TRUE ("Page Visible")) -> ()  [unwired: 1 in, 2 out]
                        }
                        frame #2 {
                          n438 = Wait (ms)(milliseconds to wait=u32 50) -> ()  [unwired: 1 out]
                        }
                        frame #3 {
                          n439 = local read "KCubeSolenoidControl"() -> (w514:refnum<k24>)
                          n440 = property class="KCubeSolenoidControl"(reference=w514, "SerialNumber"="68001425") -> (reference out=w515:refnum<k24>)  [unwired: 1 in, 1 out]
                          n441 = invoke class="KCubeSolenoidControl" method="CreateDevice"(reference=w515) -> (reference out=w516:refnum<k24>)  [unwired: 2 in, 2 out]
                          n442 = property class="KCubeSolenoidControl"(reference=w516) -> (reference out=w517:refnum<k24>, "Device"=w518:refnum<k24>)  [unwired: 1 in, 1 out]
                          n443 = invoke class="KCubeSolenoid" method="GetOperatingState"(reference=w518) -> (reference out=w519:refnum<k24>, "GetOperatingState"=w520:i32)  [unwired: 2 in, 1 out]
                          n444 = local write "KCubeSolenoidControl Reference"(w517) -> ()
                          n445 = case shown="2, Default" w520 {
                            frame 1 {
                              n446 = property on="Shutter Ctrls" class="Ring (strict)"("Value"=u16 5 ("Shutter Ctrls")) -> ()  [unwired: 2 in, 2 out]
                            }
                            frame 2, Default {
                              n447 = property on="Shutter Ctrls" class="Ring (strict)"("Value"=u16 0 ("Shutter Ctrls")) -> ()  [unwired: 2 in, 2 out]
                            }
                          }
                          n448 = local write "KCube Shutter Device Reference"(w519) -> ()
                        }
                      }
                    }
                  }
                }
                frame #1 {
                  # "Piezos objective"
                  n449 = case shown="True" "KCubes Piezo On?" {
                    tunnel: [FALSE ("Page Visible") TRUE] -> w524
                    frame False {
                      n450 = disable-structure shown="Disabled" {
                        frame Disabled {
                          n451 = control-ref of="Experimental parameters tab"() -> (w530:refnum<vi>)
                          n452 = property class="TabCtl (strict)"(reference=w530) -> ("Pages"=w533:refnum<vi>[])  [unwired: 1 in, 2 out]
                          n453 = Index Array(array=w533, index=4) -> (element=w534:refnum<vi>)
                          n454 = property class="Page"(reference=w534, "PageVis"=FALSE ("Page Visible")) -> ()  [unwired: 1 in, 2 out]
                        }
                        frame Enabled {
                        }
                      }
                    }
                    frame True {
                      n455 = stacked-sequence {
                        frame #0 {
                          n456 = local read "Log file"() -> (w538:string)
                          n457 = call "Write2LogFile.vi"("Add to log file"="Initialise communication with Objective Piezos", "Log file before"=w538, "Checkbox"=FALSE) -> ("Log file after"=w539:string)
                          n458 = local write "Log file"(w539) -> ()
                        }
                        frame #1 {
                          n459 = control-ref of="Experimental parameters tab"() -> (w543:refnum<vi>)
                          n460 = property class="TabCtl (strict)"(reference=w543, "Value"=T19."Microscope objective") -> ("Pages"=w544:refnum<vi>[])  [unwired: 1 in, 2 out]
                          n461 = Index Array(array=w544, index=4) -> (element=w545:refnum<vi>)
                          n462 = property class="Page"(reference=w545, "PageVis"=TRUE ("Page Visible")) -> ()  [unwired: 1 in, 2 out]
                        }
                        frame #2 {
                          n463 = local read "KCubePiezoControl X"() -> (w551:refnum<k24>)
                          n464 = property class="KCubePiezoControl"(reference=w551, "SerialNumber"="29502682") -> (reference out=w550:refnum<k24>)  [unwired: 1 in, 1 out]
                          n465 = invoke class="KCubePiezoControl" method="CreateDevice"(reference=w550) -> (reference out=w549:refnum<k24>)  [unwired: 2 in, 2 out]
                          n466 = property class="KCubePiezoControl"(reference=w549) -> (reference out=w548:refnum<k24>, "Device"=w547:refnum<k24>)  [unwired: 1 in, 1 out]
                          n467 = local write "KCubePiezoControl X Reference"(w548) -> ()
                          n468 = local write "KCubePiezoDevice X Reference"(w547) -> ()
                        }
                        frame #3 {
                          n469 = local read "KCubePiezoControl Y"() -> (w552:refnum<k24>)
                          n470 = property class="KCubePiezoControl"(reference=w552, "SerialNumber"="29502721") -> (reference out=w554:refnum<k24>)  [unwired: 1 in, 1 out]
                          n471 = invoke class="KCubePiezoControl" method="CreateDevice"(reference=w554) -> (reference out=w555:refnum<k24>)  [unwired: 2 in, 2 out]
                          n472 = property class="KCubePiezoControl"(reference=w555) -> (reference out=w556:refnum<k24>, "Device"=w557:refnum<k24>)  [unwired: 1 in, 1 out]
                          n473 = local write "KCubePiezoControl Y Reference"(w556) -> ()
                          n474 = local write "KCubePiezoDevice Y Reference"(w557) -> ()
                        }
                        frame #4 {
                          n475 = local read "KCubePiezoControl Z"() -> (w559:refnum<k24>)
                          n476 = property class="KCubePiezoControl"(reference=w559, "SerialNumber"="29250034") -> (reference out=w560:refnum<k24>)  [unwired: 1 in, 1 out]
                          n477 = invoke class="KCubePiezoControl" method="CreateDevice"(reference=w560) -> (reference out=w561:refnum<k24>)  [unwired: 2 in, 2 out]
                          n478 = property class="KCubePiezoControl"(reference=w561) -> (reference out=w562:refnum<k24>, "Device"=w563:refnum<k24>)  [unwired: 1 in, 1 out]
                          n479 = local write "KCubePiezoControl Z Reference"(w562) -> ()
                          n480 = local write "KCubePiezoDevice Z Reference"(w563) -> ()
                        }
                        frame #5 {
                          n481 = local read "KCubePiezoDevice Z Reference"() -> (w567:refnum<k24>)
                          n482 = call "KCube_IsActiveAndActivate.vi"("KCubePiezoDevice Z Reference"=w567) -> ("IsSetOutputVoltageActive"=→"IsSetOutputVoltageActive":bool, "reference out"=w565:refnum<k24>, "GetOutputVoltage"=→"GetOutputVoltage":dbl)  [unwired: 8 in]
                          n483 = local write "KCubePiezoDevice Z Reference"(w565) -> ()
                        }
                      }
                    }
                  }
                  n484 = control-ref of="Tab Objective Sample"() -> (w527:refnum<vi>)
                  n485 = property class="TabCtl (strict)"(reference=w527) -> ("Pages"=w526:refnum<vi>[])  [unwired: 1 in, 2 out]